vi "testDLL.vi"() -> ()   [LabVIEW 2012]
uses:
  OpenCvGlobals.vi
  <vilib>/Utility/file.llb/Read From Spreadsheet File (I64).vi
  <vilib>/Analysis/baseanly.llb/Mean (DBL).vi
  <resource>/objmgr/IMAQImage.rc
  <vilib>/Analysis/NI_AALBase.lvlib
panel:
  in  "wait after each sequence":bool
  in  "start path":path=path "E:/wingX data/keep"
  in  "minImageNumber":i32=3
  in  "default dir":bool
  in  "data folder":string="data example"
  out "mean frequency":dbl=16.816143497757846 format="%0.2f"
  out "mean dt":dbl=59.46666666666667 format="%0.2f"
  out "min dt":i32=39
  out "max dt":i32=92
  out "dt":u32=40
  out "centerYBright":dbl=324.0
  out "centerXBright":dbl=936.0
  out "rotBright":dbl=-1.1532118075075974
  out "WS":T1(plugin-control)
  in  "Image processing preferences":T2={"scale"=0.5, "elSizeImOpen"=21, "thresholdBinarizationBody"=0.5, "thresholdBinarizationWings"=0.08, "minWingArea"=20000, "quantile"=0.05, "elSizeImOpenIdent1"=15, "elSizeImOpenIdent2"=21, "thresholdBinarizationIdent"=0.65, "elSizeImHMin"=6, "raiseParImHMin"=0.33, "focus limit"=100, "maxAllowedRotation"=30.0, "elSizeImClose"=3, "numIterImClose"=3, "symmetryMinOverlapBody"=95.0, "symmetryMinOverlapWings"=80.0, "thresholdReflectionCheck"=0.99, "elSizeReflection"=7, "maxReflectionArea"=2000, "upSideDownCheck"=275.0}
  in  "isDebug":bool
  out "# image loaded":i32=14
  out "background":T1(plugin-control)
  out "return type":i32=1
  out "Image Size":cluster{"x":i32, "y":i32}={"x"=1500, "y"=600}
  out "frame":T1(plugin-control)
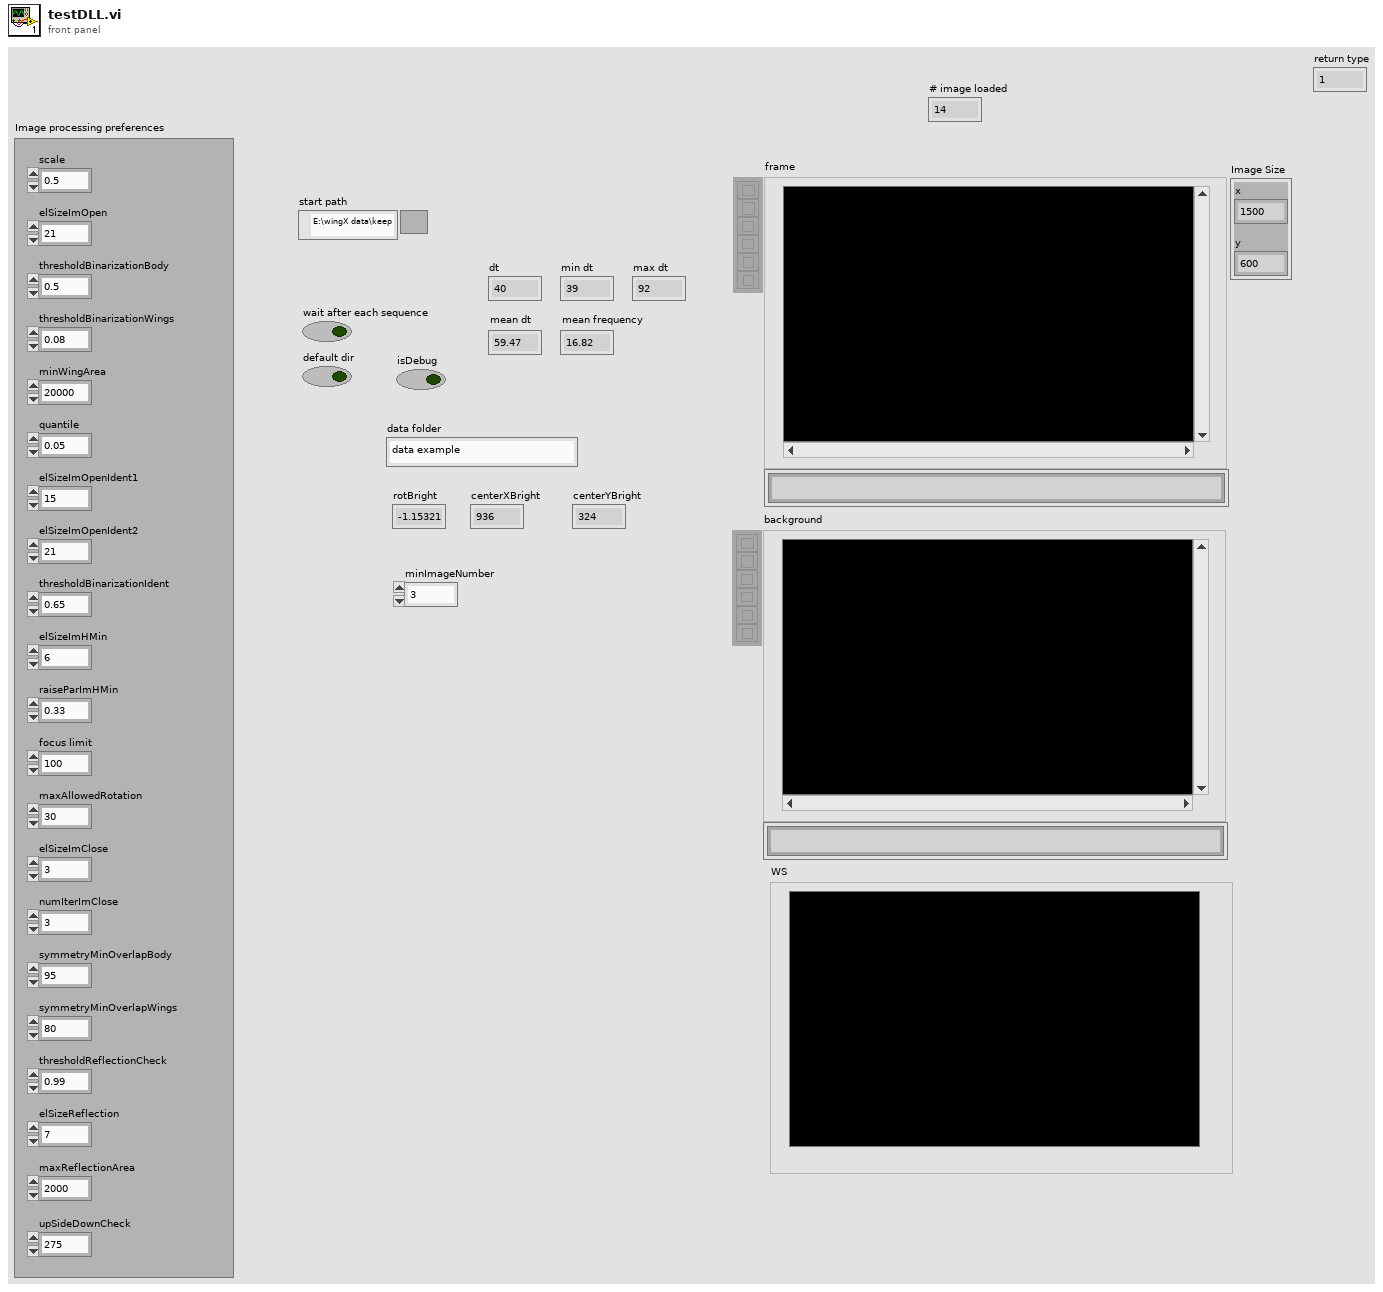
[diagram p1: front panel]
types:
  T1 = typedef "IMAQ Image.ctl" = refnum<image>
  T2 = cluster{"scale":sgl, "elSizeImOpen":i32, "thresholdBinarizationBody":sgl, "thresholdBinarizationWings":sgl, "minWingArea":i32, "quantile":sgl, "elSizeImOpenIdent1":i32, "elSizeImOpenIdent2":i32, "thresholdBinarizationIdent":sgl, "elSizeImHMin":i32, "raiseParImHMin":sgl, "focus limit":i32, "maxAllowedRotation":sgl, "elSizeImClose":i32, "numIterImClose":i32, "symmetryMinOverlapBody":sgl, "symmetryMinOverlapWings":sgl, "thresholdReflectionCheck":sgl, "elSizeReflection":i32, "maxReflectionArea":i32, "upSideDownCheck":sgl}
  T3 = typedef "Image Type" = u32
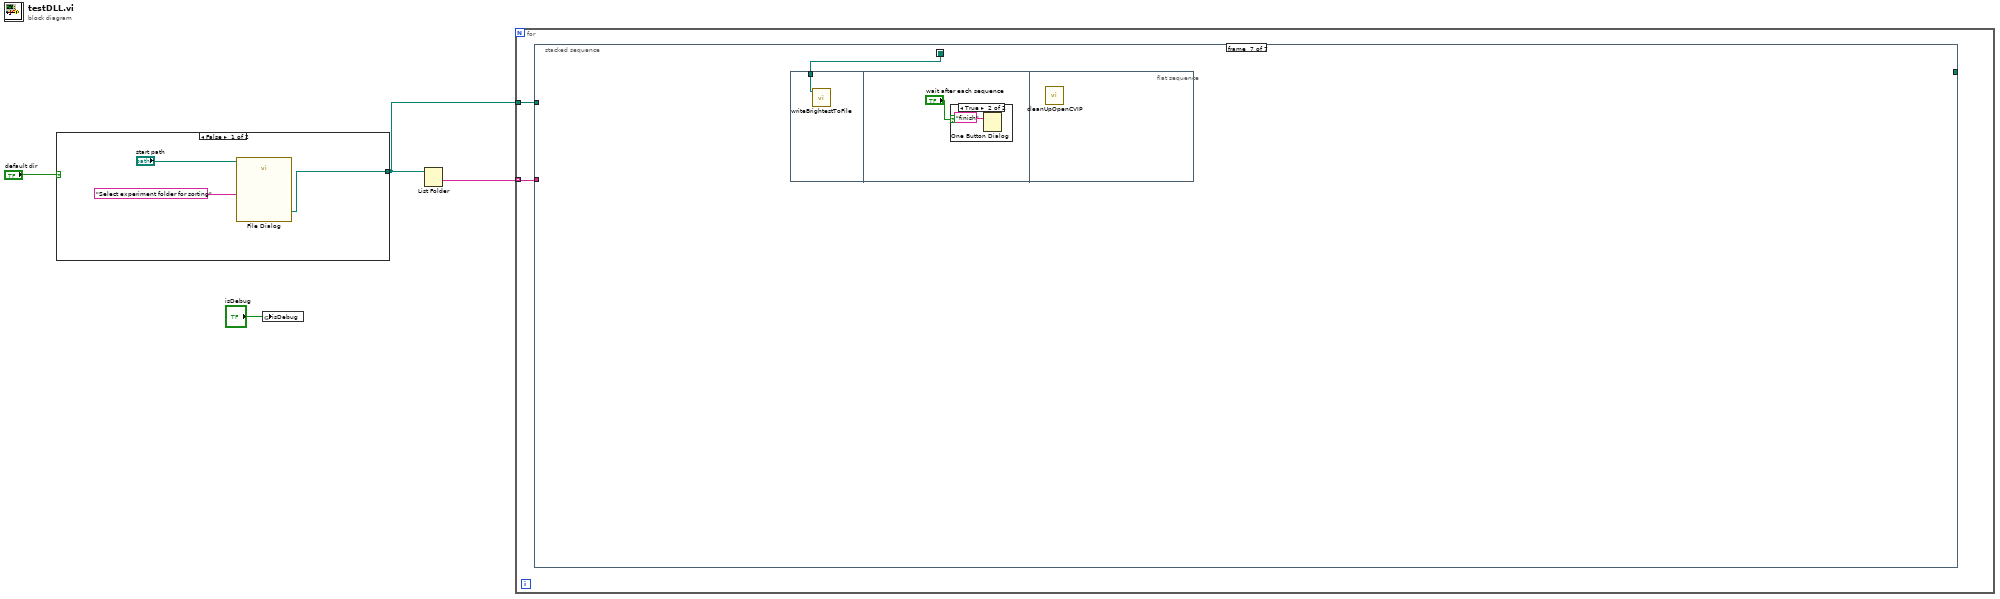
[diagram p0: block diagram]
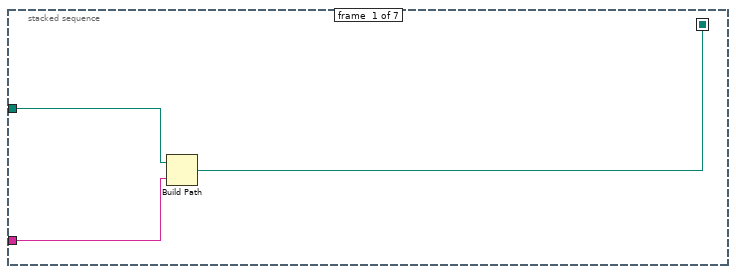
[diagram p2: hidden frame]
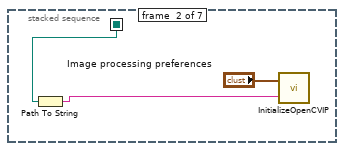
[diagram p3: hidden frame]
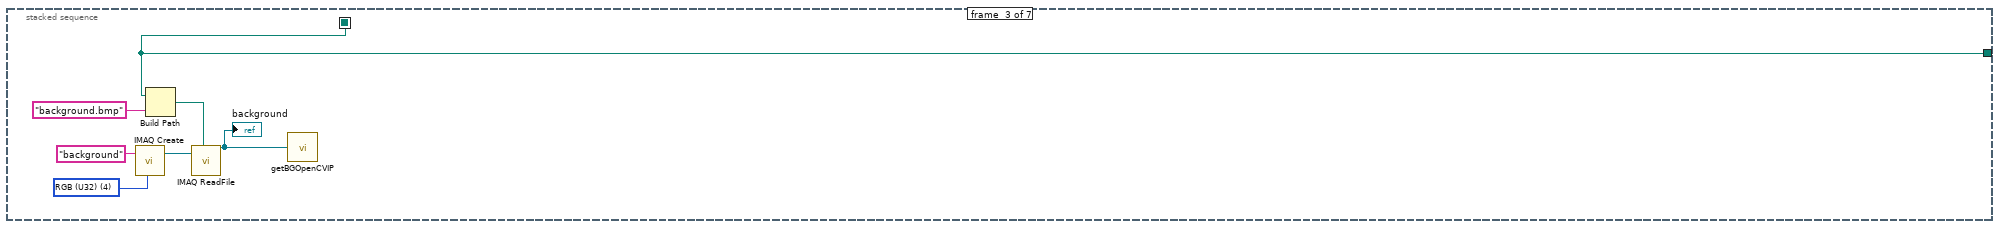
[diagram p4: hidden frame]
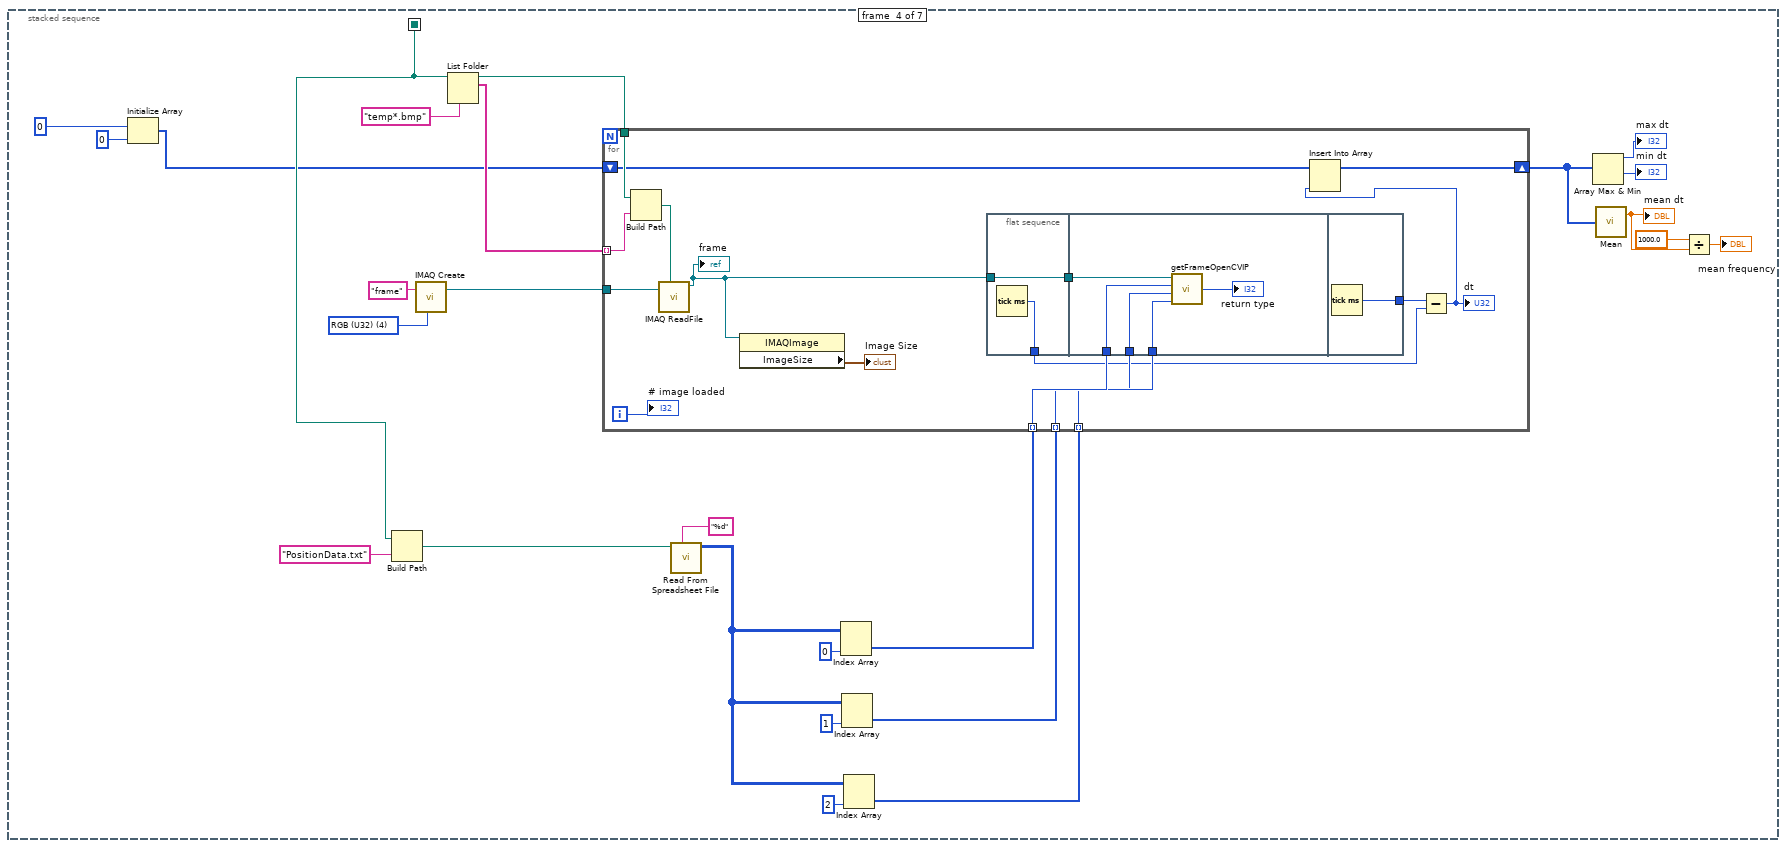
[diagram p5: hidden frame]
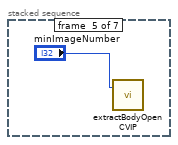
[diagram p6: hidden frame]
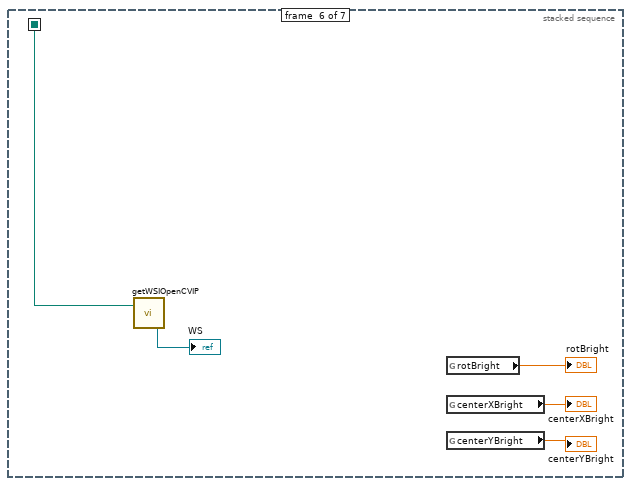
[diagram p7: hidden frame]
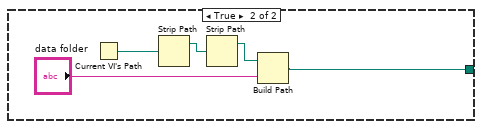
[diagram p9: hidden frame]
diagram:
  n1 = case shown="False" "default dir" {
    tunnel: [w6 w8] -> w2
    frame False {
      n2 = call "File Dialog"("start path"="start path", "prompt"="Select experiment folder for sorting") -> ("selected path"=w6:path)  [unwired: 10 in, 3 out]
    }
    frame True {
      n3 = Current VI's Path() -> (path=w11:path)
      n4 = Strip Path(path=w11) -> (stripped path=w10:path)  [unwired: 1 out]
      n5 = Strip Path(path=w10) -> (stripped path=w9:path)  [unwired: 1 out]
      n6 = Build Path(base path=w9, name or relative path="data folder") -> (appended path=w8:path)
    }
  }
  n7 = global write "OpenCvGlobals.vi" "isDebug"("isDebug") -> ()
  n8 = List Folder(path=w2) -> (folder names=w1:string[])  [unwired: 3 in, 3 out]
  n9 = for {
    tunnel: w2 -> [w14]
    tunnel: w1 -> [w13] mode=indexing
    n10 = stacked-sequence {
      seq-local: [w16 _ _ _ _ _ _] -> [_ w20 w21 w37 _ w79 w84]
      tunnel: [_ _ w21 _ _ _ _] -> _
      tunnel: w14 -> [w17 _ _ _ _ _ _]
      tunnel: w13 -> [w15 _ _ _ _ _ _]
      frame #0 {
        n11 = Build Path(base path=w17, name or relative path=w15) -> (appended path=w16:path)
      }
      frame #1 {
        n12 = Path To String(path=w20) -> (string=w19:string)
        n13 = call "InitializeOpenCVIP.vi"("dataDirectory"=w19, "Image processing preferences"="Image processing preferences") -> ()  [unwired: 1 out]
      }
      frame #2 {
        w26 = T3 4 items=["Grayscale (U8)", "Grayscale (I16)", "Grayscale (SGL)", "Complex (CSG)", "RGB (U32)", "HSL (U32)", "RGB (U64)", "Grayscale (U16)"] ("Image Type")
        n14 = call "IMAQ Create"("Image Name"="background", "Image Type"=w26) -> ("New Image"=w24:T1)  [unwired: 2 in, 2 out]
        n15 = Build Path(base path=w21, name or relative path="background.bmp") -> (appended path=w22:path)
        n16 = call "IMAQ ReadFile"("File Path"=w22, "Image"=w24) -> ("Image Out"=w27:T1)  [unwired: 3 in, 6 out]
        "background" <- w27
        n17 = call "getBGOpenCVIP.vi"("Image"=w27) -> ()  [unwired: 1 out]
      }
      frame #3 {
        w40 = T3 4 items=["Grayscale (U8)", "Grayscale (I16)", "Grayscale (SGL)", "Complex (CSG)", "RGB (U32)", "HSL (U32)", "RGB (U64)", "Grayscale (U16)"] ("Image Type")
        n18 = Initialize Array(0 ("element"), 0 ("dimension size")) -> (w35:i32[])
        n19 = Build Path(base path=w37, name or relative path="PositionData.txt") -> (appended path=w53:path)
        n20 = call "IMAQ Create"("Image Name"="frame", "Image Type"=w40) -> ("New Image"=w38:T1)  [unwired: 2 in, 2 out]
        n21 = List Folder(path=w37, pattern="temp*.bmp") -> (path out=w43:path, filenames=w42:string[])  [unwired: 2 in, 2 out]
        n22 = call-poly <vilib>:"Read From Spreadsheet File.vi"("format (%d)"="%d", "file path (dialog if empty)"=w53) -> ("all rows"=w52:i64[][])  [unwired: 5 in, 4 out]
        n23 = Index Array(array=w52, index (col)=0 ("disabled index (col)")) -> (element=w45:i64[])  [unwired: 1 in]
        n24 = Index Array(array=w52, index (col)=1 ("disabled index (col)")) -> (element=w46:i64[])  [unwired: 1 in]
        n25 = Index Array(array=w52, index (col)=2 ("disabled index (col)")) -> (element=w47:i64[])  [unwired: 1 in]
        n26 = for {
          tunnel: w38 -> [w69]
          tunnel: w42 -> [w64] mode=indexing
          tunnel: w43 -> [w66]
          tunnel: w45 -> [w63] mode=indexing
          tunnel: w46 -> [w61] mode=indexing
          tunnel: w47 -> [w62] mode=indexing
          shift-right: [w55] -> w31
          shift-left: w35 -> [w56]
          i -> [w67]
          n27 = Build Path(base path=w66, name or relative path=w64) -> (appended path=w65:path)
          n28 = call "IMAQ ReadFile"("File Path"=w65, "Image"=w69) -> ("Image Out"=w60:T1)  [unwired: 3 in, 6 out]
          "frame" <- w60
          n29 = property class="IMAQImage"(reference=w60) -> ("ImageSize"=→"Image Size":cluster{"x":i32, "y":i32})  [unwired: 1 in, 2 out]
          n30 = flat-sequence {
            tunnel: w60 -> [w71]
            tunnel: [w71] -> w59
            tunnel: [w70] -> w57
            tunnel: w63 -> [w76]
            tunnel: w62 -> [w75]
            tunnel: w61 -> [w74]
            tunnel: w59 -> [w73]
            tunnel: [w77] -> w58
            frame #0 {
              n31 = Tick Count (ms)() -> (millisecond timer value=w70:u32)
            }
            frame #1 {
              n32 = call "getFrameOpenCVIP.vi"("cropY"=w75, "cropX"=w74, "frameNumber"=w76, "Image"=w73) -> ("return type"=→"return type":i32)
            }
            frame #2 {
              n33 = Tick Count (ms)() -> (millisecond timer value=w77:u32)
            }
          }
          n34 = Subtract(x=w58, y=w57) -> (x-y=w54:u32)
          "dt" <- w54
          n35 = Insert Into Array(array=w56, new element=w54) -> (w55:i32[])  [unwired: 1 in]
          "# image loaded" <- w67
        }
        n36 = Array Max & Min(array=w31) -> (max value=→"max dt":i32, min value=→"min dt":i32)  [unwired: 2 out]
        n37 = call-poly <vilib>:"Mean.vi"("X"=w31) -> ("mean"=w29:dbl)  [unwired: 1 out]
        "mean dt" <- w29
        n38 = Divide(x=1000.0, y=w29) -> (x/y=→"mean frequency":dbl)
      }
      frame #4 {
        n39 = call "extractBodyOpenCVIP.vi"("minImageNumber"="minImageNumber") -> ()  [unwired: 2 in, 1 out]
      }
      frame #5 {
        n40 = call "getWSIOpenCVIP.vi"("File Path"=w79) -> ("Image Dst Out"=→"WS":T1)  [unwired: 1 in, 1 out]
        n41 = global read "OpenCvGlobals.vi" "rotBright"() -> (→"rotBright":dbl)
        n42 = global read "OpenCvGlobals.vi" "centerXBright"() -> (→"centerXBright":dbl)
        n43 = global read "OpenCvGlobals.vi" "centerYBright"() -> (→"centerYBright":dbl)
      }
      frame #6 {
        n44 = flat-sequence {
          tunnel: w84 -> [w85]
          frame #0 {
            n45 = call "writeBrightestToFile.vi"("base path"=w85) -> ()  [unwired: 11 in]
          }
          frame #1 {
            n46 = case shown="True" "wait after each sequence" {
              frame False {
              }
              frame True {
                n47 = One Button Dialog(message="finish") -> ()  [unwired: 1 in, 1 out]
              }
            }
          }
          frame #2 {
            n48 = call "cleanUpOpenCVIP.vi"() -> ()  [unwired: 4 in, 1 out]
          }
        }
      }
    }
  }
